vi "TLB Native Dynamic Events ver 0.26.vi"() -> ()   [LabVIEW 2018] (continued)
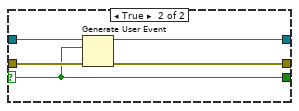
[diagram p2: hidden frame]
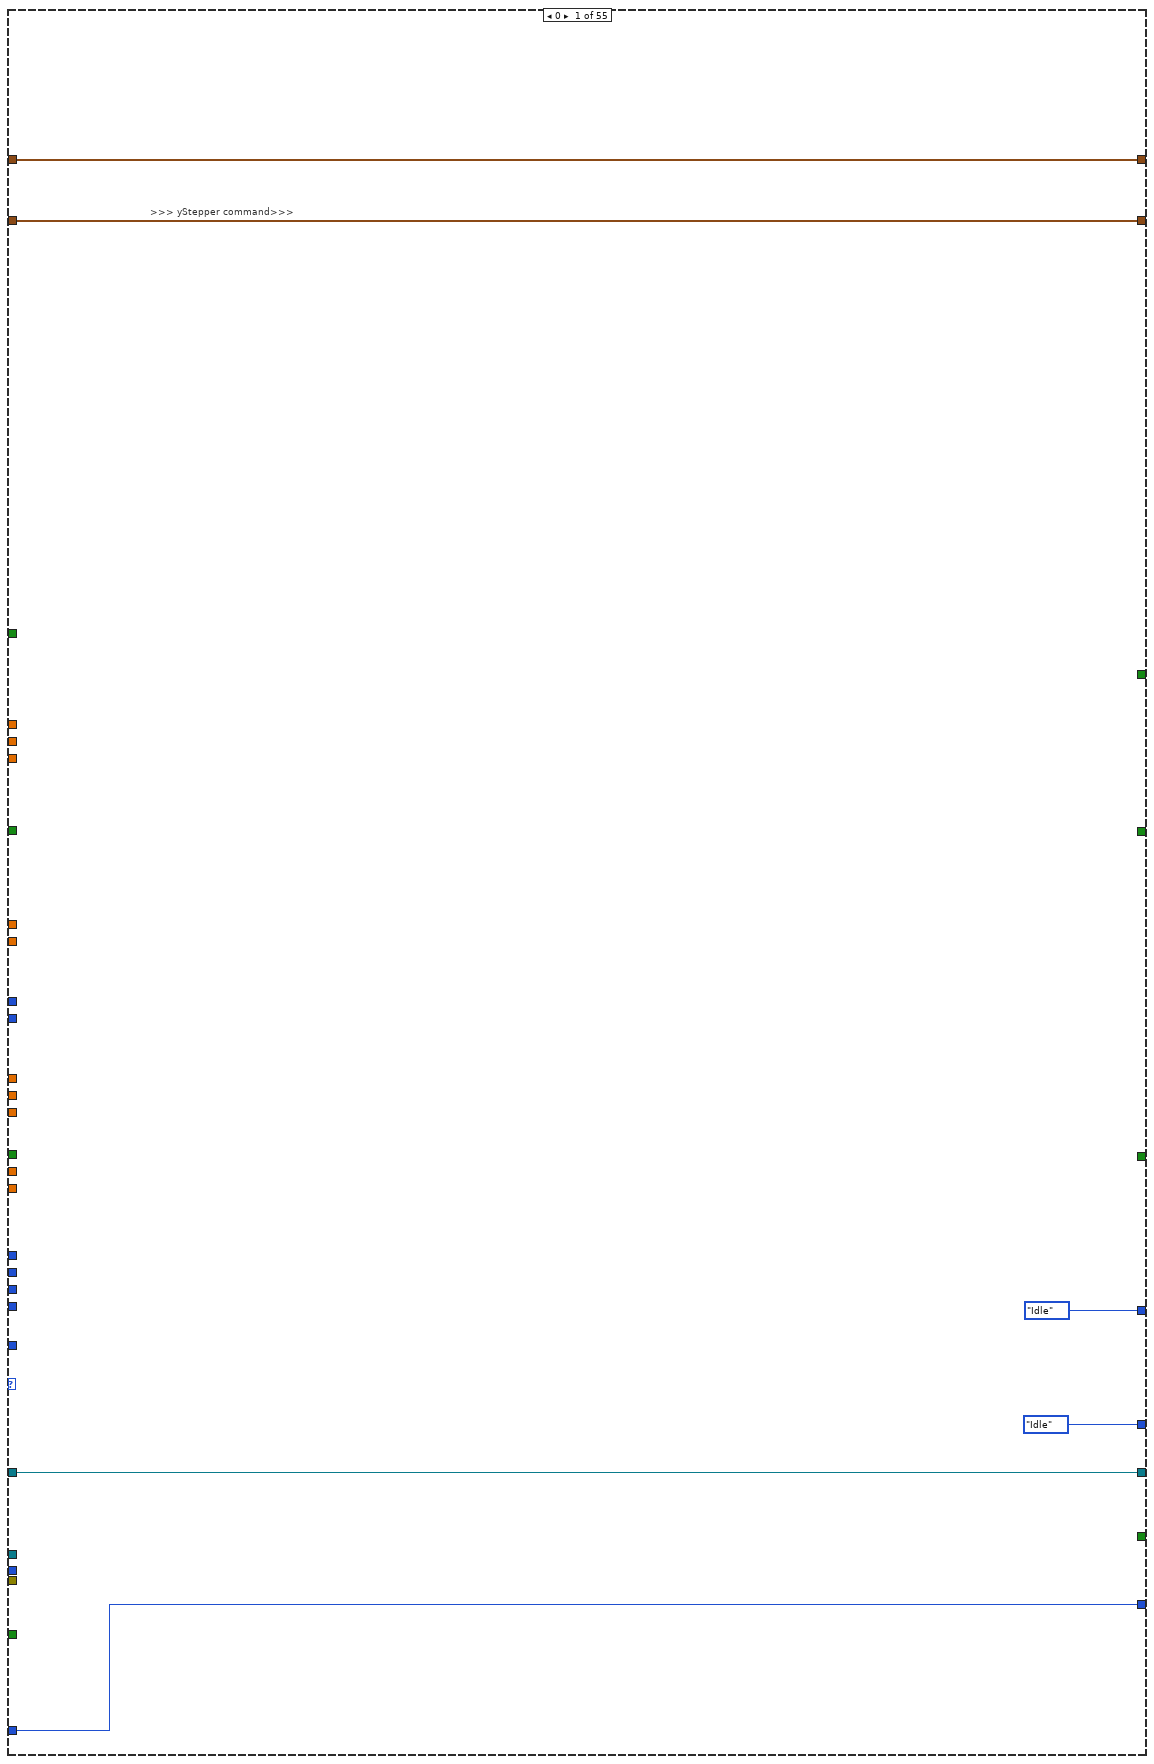
[diagram p5: hidden frame]
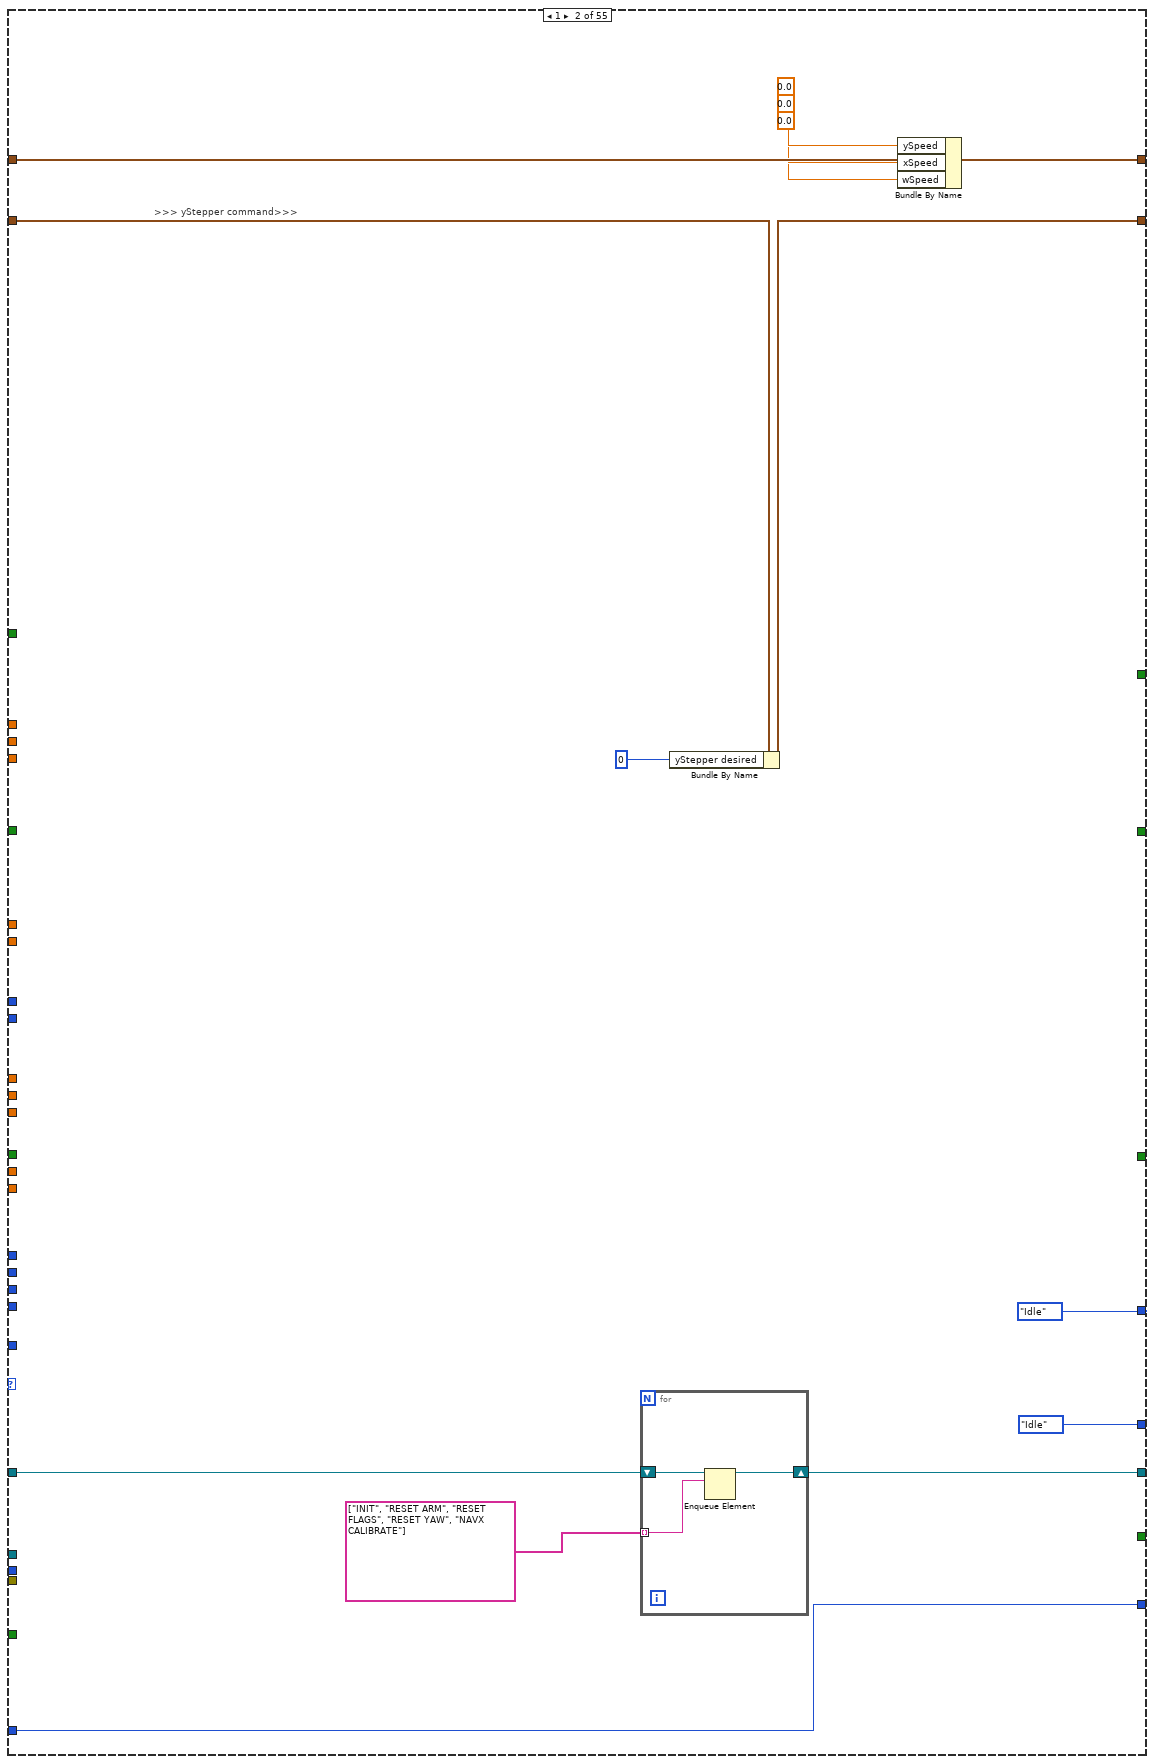
[diagram p6: hidden frame]
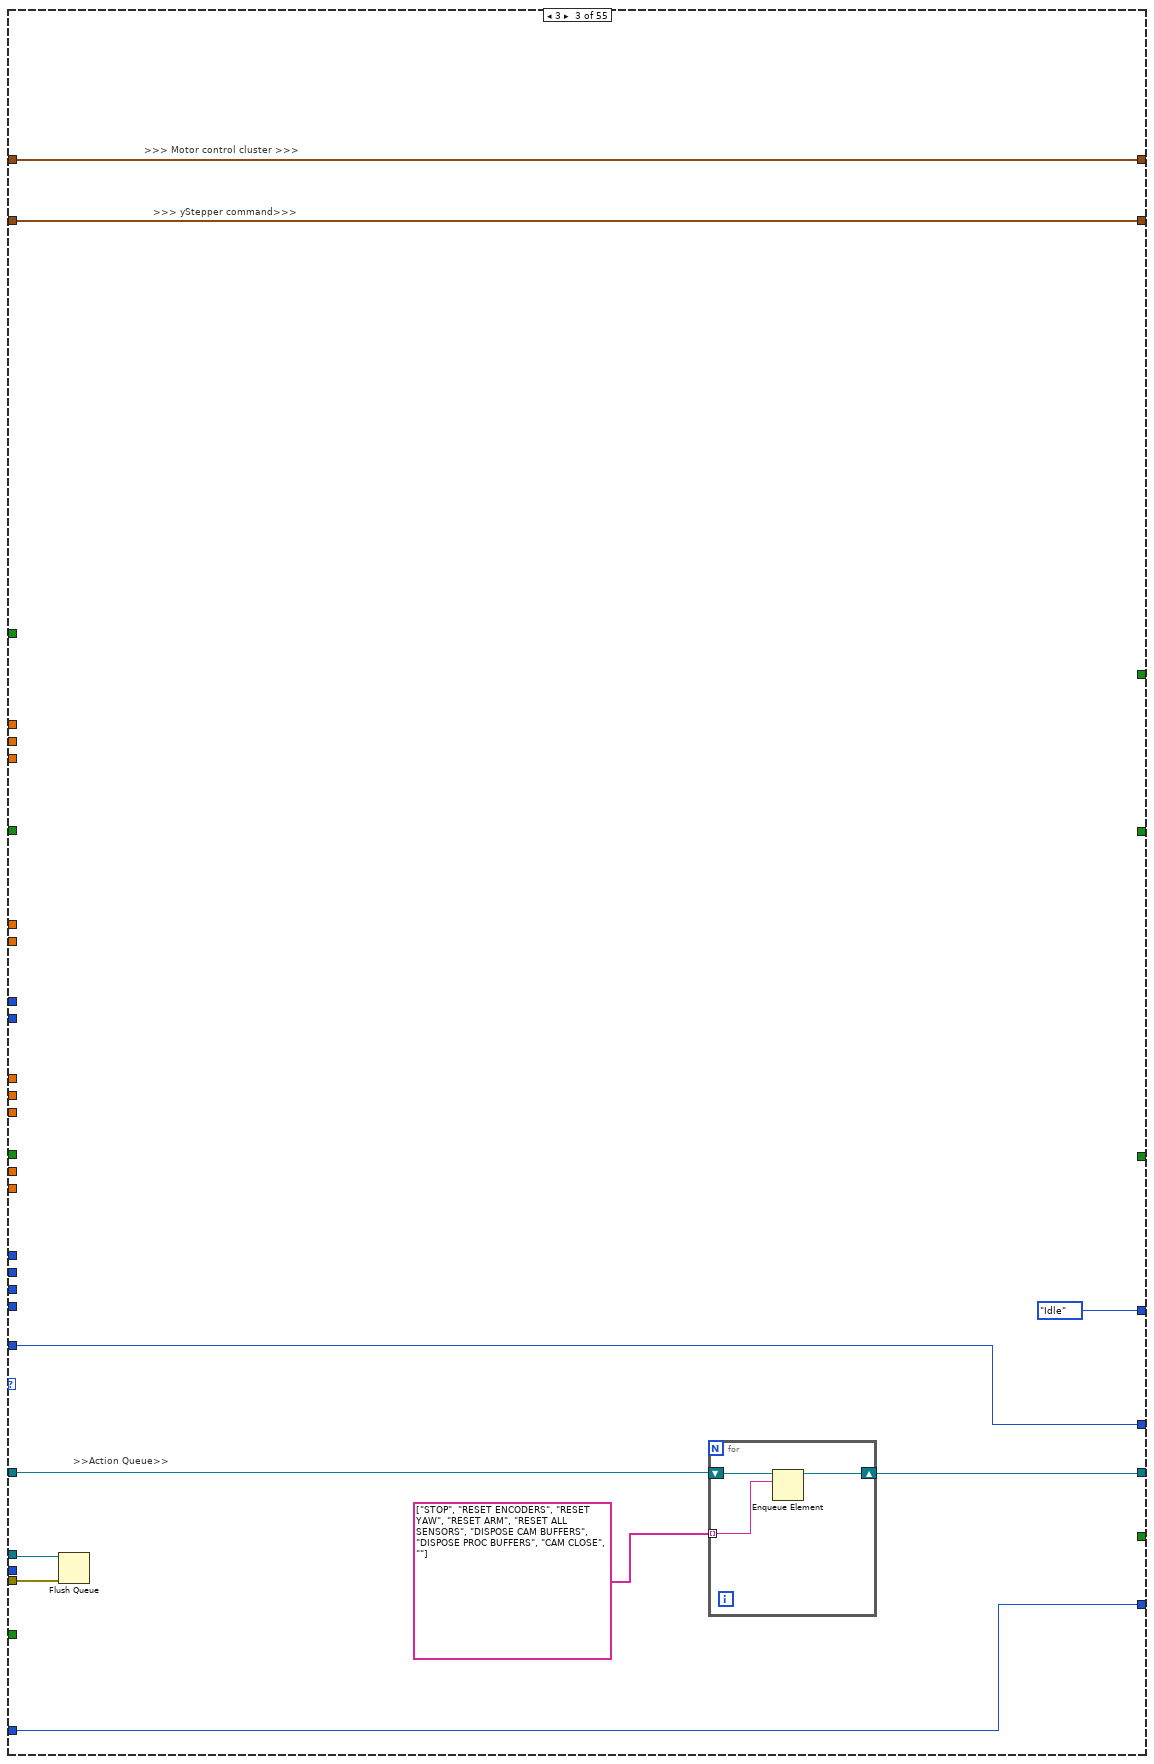
[diagram p7: hidden frame]
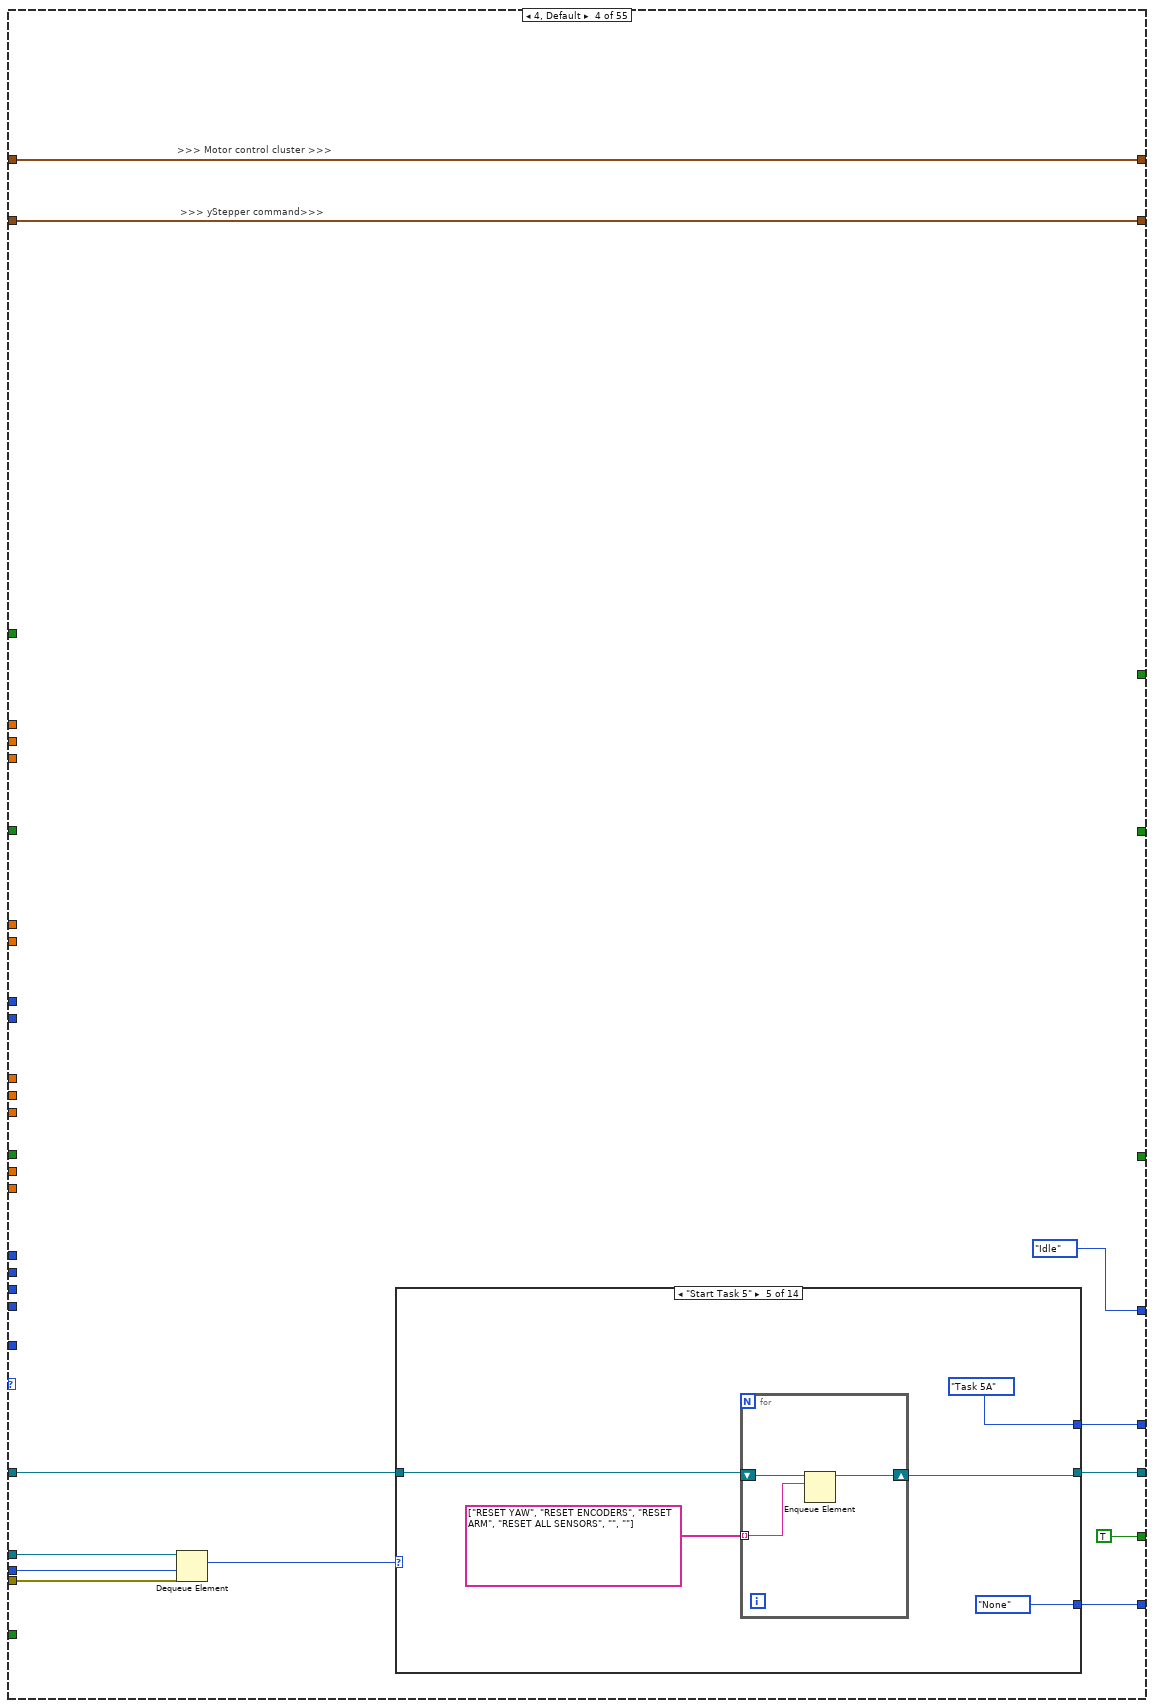
[diagram p8: hidden frame]
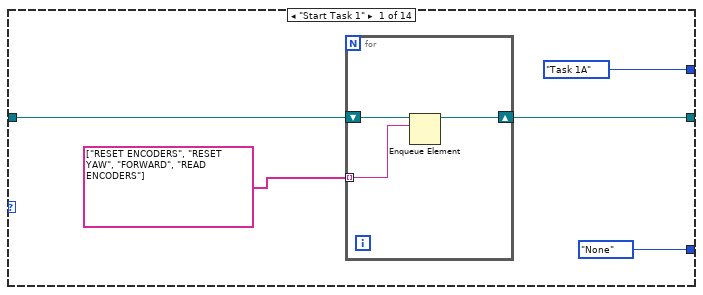
[diagram p9: hidden frame]
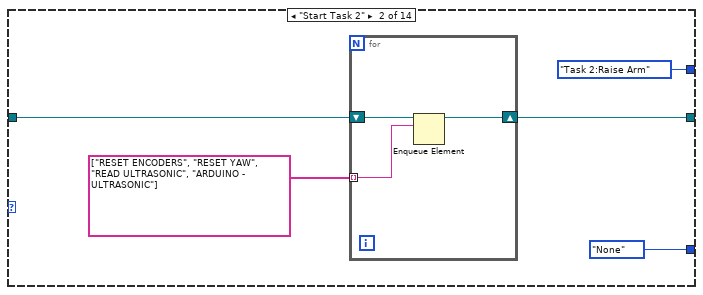
[diagram p10: hidden frame]
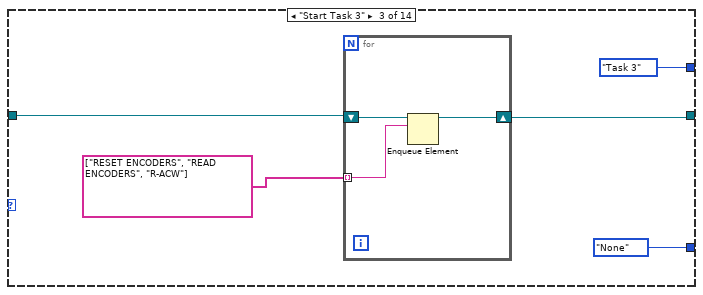
[diagram p11: hidden frame]
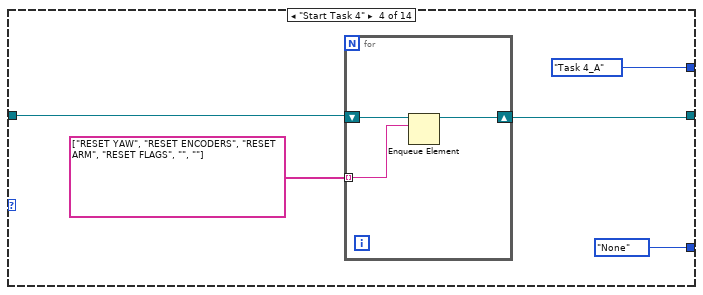
[diagram p12: hidden frame]
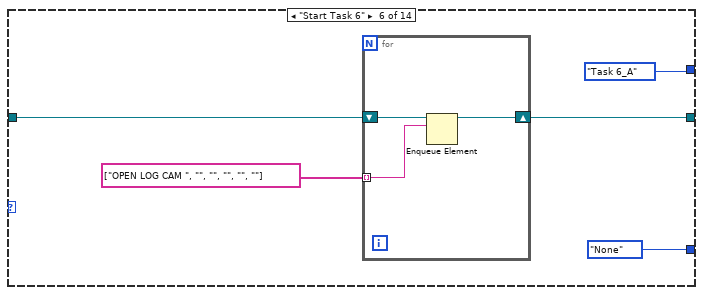
[diagram p13: hidden frame]
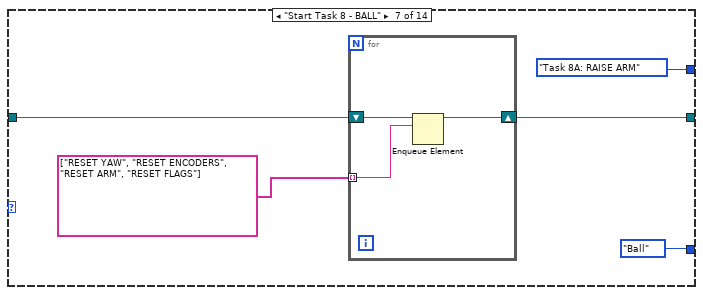
[diagram p14: hidden frame]
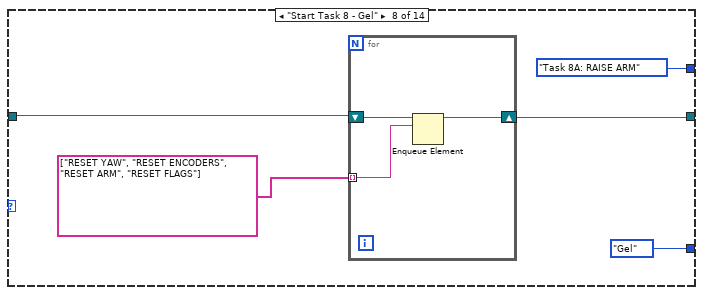
[diagram p15: hidden frame]
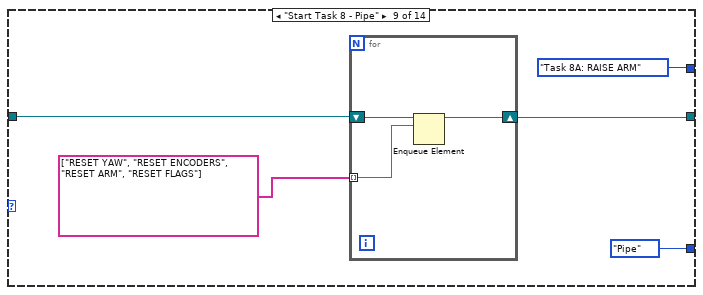
[diagram p16: hidden frame]
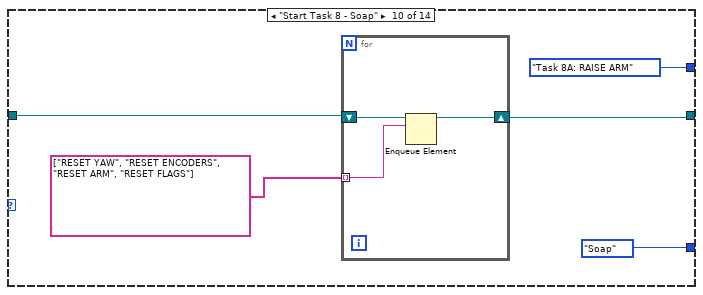
[diagram p17: hidden frame]
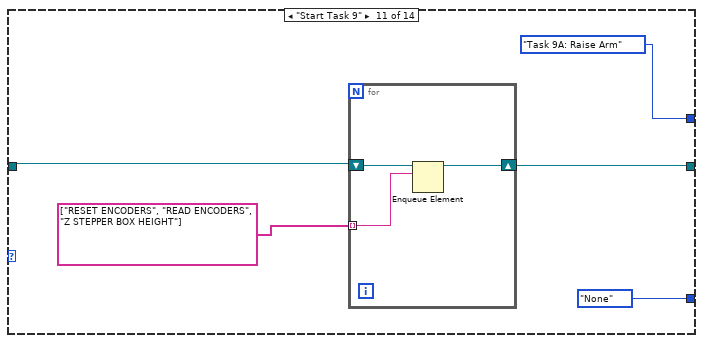
[diagram p18: hidden frame]
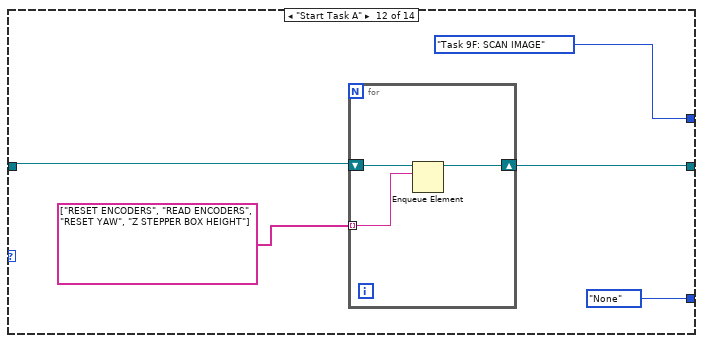
[diagram p19: hidden frame]
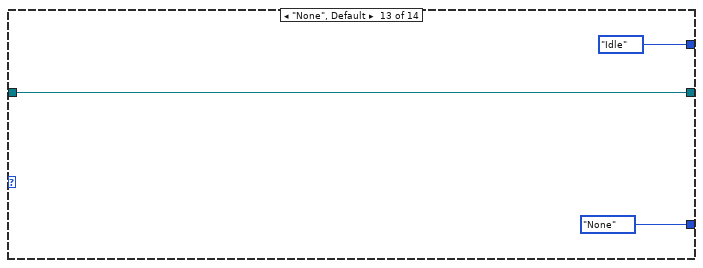
[diagram p20: hidden frame]
                      shift-left: w2521 -> [w2524]
                      n813 = Enqueue Element(queue=w2524, element=w2523) -> (queue out=w2525:refnum<queue>)  [unwired: 2 in, 2 out]
                    }
                  }
                  frame True {
                    n814 = for {
                      shift-right: [w2530] -> w2527
                      shift-left: w2528 -> [w2531]
                      tunnel: string[] ["STOP", "RESET ENCODERS", "RESET YAW", "OPEN LIFE CAM", "SET TIMER 2", "RESET FLAGS"] -> [w2529] mode=indexing
                      n815 = Enqueue Element(queue=w2531, element=w2529) -> (queue out=w2530:refnum<queue>)  [unwired: 2 in, 2 out]
                    }
                  }
                }
                n816 = Or(x=w2511, y=w2510) -> (x .or. y?=w2509:bool)
                n817 = Select(t=State_Type_Definitions,_for_0.26g_versions_and_later_2."True Stop" ("Enum"), s=w2510, f=State_Type_Definitions."Task 9N: SCAN IMAGE" ("Enum")) -> (s? t:f=w2512:u16)
                n818 = Select(t=w2512, s=w2509, f=State_Type_Definitions,_for_0.26g_versions_and_later_2."Task 9M: MOVE RIGHT" ("Enum")) -> (s? t:f=w2518:u16)
              }
              frame "Exit" {
                n819 = for {
                  shift-right: [w2538] -> w2535
                  shift-left: w2534 -> [w2539]
                  tunnel: string[] ["STOP", "RESET ENCODERS", "RESET YAW", "ARDUINO MODE 0"] -> [w2537] mode=indexing
                  n820 = Enqueue Element(queue=w2539, element=w2537) -> (queue out=w2538:refnum<queue>)  [unwired: 2 in, 2 out]
                }
              }
            }
          }
          frame 51 {
            # ">> Manual override >>"
            n821 = Dequeue Element(queue=w2548, timeout in ms (-1)=w2547, error in (no error)=w2546) -> (element=w2549:T8)  [unwired: 3 out]
            n822 = case shown="\"Start Task 1\", Default" w2549 {
              tunnel: [w2563 State_Type_Definitions,_for_0.26g_versions_and_later_2."True Stop" ("Enum")] -> w2541
              tunnel: [w2561 w2579] -> w2540
              tunnel: w2544 -> [w2560 w2576]
              tunnel: w2545 -> [w2554 _]
              tunnel: [State_Type_Definitions,_for_0.26g_versions_and_later_2."Idle" ("Enum") State_Type_Definitions,_for_0.26g_versions_and_later_2."Shutdown" ("Enum")] -> w2542
              tunnel: w2543 -> [w2553 _]
              frame "Start Task 1", Default {
                # ">> WIill proceed to part ii if not manual override >>"
                # ">>If ENABLE or Trigger is set to true>>"
                n823 = Or(x=w2553, y=w2554) -> (x .or. y?=w2555:bool)
                n824 = case shown="False" w2553 {
                  tunnel: [w2566 w2572] -> w2561
                  tunnel: w2560 -> [w2565 w2571]
                  frame False {
                    n825 = for {
                      shift-right: [w2568] -> w2566
                      shift-left: w2565 -> [w2569]
                      tunnel: string[] ["CAM ACQ", "START TIMER"] ("element") -> [w2567] mode=indexing
                      n826 = Enqueue Element(queue=w2569, element=w2567) -> (queue out=w2568:refnum<queue>)  [unwired: 2 in, 2 out]
                    }
                  }
                  frame True {
                    n827 = for {
                      shift-right: [w2574] -> w2572
                      shift-left: w2571 -> [w2575]
                      tunnel: string[] ["CLOSE CAM", "SET TIMER 5", "", "", "", ""] -> [w2573] mode=indexing
                      n828 = Enqueue Element(queue=w2575, element=w2573) -> (queue out=w2574:refnum<queue>)  [unwired: 2 in, 2 out]
                    }
                  }
                }
                n829 = Select(t=State_Type_Definitions,_for_0.26g_versions_and_later_2."True Stop" ("Enum"), s=w2554, f=State_Type_Definitions."Task 9O: PROCESS COLOUR" ("Enum")) -> (s? t:f=w2557:u16)
                n830 = Select(t=w2557, s=w2555, f=State_Type_Definitions."Task 9N: SCAN IMAGE" ("Enum")) -> (s? t:f=w2563:u16)
              }
              frame "Exit" {
                n831 = for {
                  shift-right: [w2582] -> w2579
                  shift-left: w2576 -> [w2583]
                  tunnel: string[] ["STOP", "RESET ENCODERS", "RESET YAW", ""] -> [w2581] mode=indexing
                  n832 = Enqueue Element(queue=w2583, element=w2581) -> (queue out=w2582:refnum<queue>)  [unwired: 2 in, 2 out]
                }
              }
            }
          }
          frame 52 {
            # ">> Item Selection Bias >>"
            n833 = Dequeue Element(queue=w2591, timeout in ms (-1)=w2590, error in (no error)=w2589) -> (element=w2593:T8)  [unwired: 3 out]
            n834 = case shown="\"Start Task 1\", Default" w2593 {
              tunnel: w2584 -> [w2599 _]
              tunnel: [w2606 State_Type_Definitions,_for_0.26g_versions_and_later_2."True Stop" ("Enum")] -> w2587
              tunnel: w2588 -> [w2598 _]
              tunnel: w2592 -> [w2605 w2622]
              tunnel: [w2604 w2623] -> w2586
              tunnel: [State_Type_Definitions,_for_0.26g_versions_and_later_2."Idle" ("Enum") State_Type_Definitions,_for_0.26g_versions_and_later_2."Shutdown" ("Enum")] -> w2585
              frame "Start Task 1", Default {
                n835 = case shown="False" w2599 {
                  tunnel: w2605 -> [w2609 w2616]
                  tunnel: [w2610 w2615] -> w2604
                  frame False {
                    n836 = for {
                      tunnel: string[] ["START TIMER", "COLOUR PROCESSING", ""] ("element") -> [w2611] mode=indexing
                      shift-right: [w2613] -> w2610
                      shift-left: w2609 -> [w2612]
                      n837 = Enqueue Element(queue=w2612, element=w2611) -> (queue out=w2613:refnum<queue>)  [unwired: 2 in, 2 out]
                    }
                  }
                  frame True {
                    n838 = for {
                      shift-right: [w2618] -> w2615
                      shift-left: w2616 -> [w2619]
                      tunnel: string[] ["CLOSE CAM", "DISPOSE BUFFERS", "RESET ENCODERS", "RESET YAW", "RESET FLAGS", ""] -> [w2617] mode=indexing
                      n839 = Enqueue Element(queue=w2619, element=w2617) -> (queue out=w2618:refnum<queue>)  [unwired: 2 in, 2 out]
                    }
                  }
                }
                n840 = Or(x=w2599, y=w2598) -> (x .or. y?=w2597:bool)
                n841 = Select(t=State_Type_Definitions,_for_0.26g_versions_and_later_2."True Stop" ("Enum"), s=w2598, f=State_Type_Definitions."Task 9P: MOVE RIGHT" ("Enum")) -> (s? t:f=w2600:u16)
                n842 = Select(t=w2600, s=w2597, f=State_Type_Definitions."Task 9O: PROCESS COLOUR" ("Enum")) -> (s? t:f=w2606:u16)
              }
              frame "Exit" {
                n843 = for {
                  shift-right: [w2626] -> w2623
                  shift-left: w2622 -> [w2627]
                  tunnel: string[] ["STOP", "RESET ENCODERS", "RESET YAW", "ARDUINO MODE 0"] -> [w2625] mode=indexing
                  n844 = Enqueue Element(queue=w2627, element=w2625) -> (queue out=w2626:refnum<queue>)  [unwired: 2 in, 2 out]
                }
              }
            }
          }
          frame 53 {
            # ">> Item Selection Bias >>"
            n845 = Dequeue Element(queue=w2633, timeout in ms (-1)=w2632, error in (no error)=w2631) -> (element=w2641:T8)  [unwired: 3 out]
            n846 = Greater?(x=w2629, y=50.0) -> (0:w2639:bool)
            n847 = And(x=w2628, y=w2639) -> (x .and. y?=w2640:bool)
            n848 = case shown="\"Start Task 1\", Default" w2641 {
              tunnel: w2640 -> [w2647 _]
              tunnel: [w2654 State_Type_Definitions,_for_0.26g_versions_and_later_2."True Stop" ("Enum")] -> w2636
              tunnel: w2630 -> [w2646 _]
              tunnel: w2634 -> [w2653 w2670]
              tunnel: [w2652 w2671] -> w2635
              tunnel: [State_Type_Definitions,_for_0.26g_versions_and_later_2."Idle" ("Enum") State_Type_Definitions,_for_0.26g_versions_and_later_2."Shutdown" ("Enum")] -> w2637
              frame "Start Task 1", Default {
                n849 = case shown="False" w2647 {
                  tunnel: w2653 -> [w2657 w2664]
                  tunnel: [w2658 w2663] -> w2652
                  frame False {
                    n850 = for {
                      tunnel: string[] ["READ LINE SENSOR", "READ NAVX", "RIGHT", "READ ENCODERS"] ("element") -> [w2659] mode=indexing
                      shift-right: [w2661] -> w2658
                      shift-left: w2657 -> [w2660]
                      n851 = Enqueue Element(queue=w2660, element=w2659) -> (queue out=w2661:refnum<queue>)  [unwired: 2 in, 2 out]
                    }
                  }
                  frame True {
                    n852 = for {
                      shift-right: [w2666] -> w2663
                      shift-left: w2664 -> [w2667]
                      tunnel: string[] ["STOP", "RESET ENCODERS", "RESET YAW", "OPEN LIFE CAM", "SET TIMER 2", "RESET FLAGS"] -> [w2665] mode=indexing
                      n853 = Enqueue Element(queue=w2667, element=w2665) -> (queue out=w2666:refnum<queue>)  [unwired: 2 in, 2 out]
                    }
                  }
                }
                n854 = Or(x=w2647, y=w2646) -> (x .or. y?=w2645:bool)
                n855 = Select(t=State_Type_Definitions,_for_0.26g_versions_and_later_2."True Stop" ("Enum"), s=w2646, f=State_Type_Definitions."Task 9Q: SCAN IMAGE" ("Enum")) -> (s? t:f=w2648:u16)
                n856 = Select(t=w2648, s=w2645, f=State_Type_Definitions."Task 9P: MOVE RIGHT" ("Enum")) -> (s? t:f=w2654:u16)
              }
              frame "Exit" {
                n857 = for {
                  shift-right: [w2674] -> w2671
                  shift-left: w2670 -> [w2675]
                  tunnel: string[] ["STOP", "RESET ENCODERS", "RESET YAW", "ARDUINO MODE 0"] -> [w2673] mode=indexing
                  n858 = Enqueue Element(queue=w2675, element=w2673) -> (queue out=w2674:refnum<queue>)  [unwired: 2 in, 2 out]
                }
              }
            }
          }
          frame 54 {
            # ">> Manual override >>"
            n859 = Dequeue Element(queue=w2684, timeout in ms (-1)=w2683, error in (no error)=w2682) -> (element=w2685:T8)  [unwired: 3 out]
            n860 = case shown="\"Start Task 1\", Default" w2685 {
              tunnel: [w2699 State_Type_Definitions,_for_0.26g_versions_and_later_2."True Stop" ("Enum")] -> w2677
              tunnel: [w2697 w2715] -> w2676
              tunnel: w2680 -> [w2696 w2712]
              tunnel: w2681 -> [w2690 _]
              tunnel: [State_Type_Definitions,_for_0.26g_versions_and_later_2."Idle" ("Enum") State_Type_Definitions,_for_0.26g_versions_and_later_2."Shutdown" ("Enum")] -> w2678
              tunnel: w2679 -> [w2689 _]
              frame "Start Task 1", Default {
                # ">> WIill proceed to part ii if not manual override >>"
                # ">>If ENABLE or Trigger is set to true>>"
                n861 = Or(x=w2689, y=w2690) -> (x .or. y?=w2691:bool)
                n862 = case shown="False" w2689 {
                  tunnel: [w2702 w2708] -> w2697
                  tunnel: w2696 -> [w2701 w2707]
                  frame False {
                    n863 = for {
                      shift-right: [w2704] -> w2702
                      shift-left: w2701 -> [w2705]
                      tunnel: string[] ["CAM ACQ", "START TIMER"] ("element") -> [w2703] mode=indexing
                      n864 = Enqueue Element(queue=w2705, element=w2703) -> (queue out=w2704:refnum<queue>)  [unwired: 2 in, 2 out]
                    }
                  }
                  frame True {
                    n865 = for {
                      shift-right: [w2710] -> w2708
                      shift-left: w2707 -> [w2711]
                      tunnel: string[] ["CLOSE CAM", "SET TIMER 5", "", "", "", ""] -> [w2709] mode=indexing
                      n866 = Enqueue Element(queue=w2711, element=w2709) -> (queue out=w2710:refnum<queue>)  [unwired: 2 in, 2 out]
                    }
                  }
                }
                n867 = Select(t=State_Type_Definitions,_for_0.26g_versions_and_later_2."True Stop" ("Enum"), s=w2690, f=State_Type_Definitions,_for_0.26g_versions_and_later_2."Task 9R: PROCESS COLOUR" ("Enum")) -> (s? t:f=w2693:T16)
                n868 = Select(t=w2693, s=w2691, f=State_Type_Definitions."Task 9Q: SCAN IMAGE" ("Enum")) -> (s? t:f=w2699:u16)
              }
              frame "Exit" {
                n869 = for {
                  shift-right: [w2718] -> w2715
                  shift-left: w2712 -> [w2719]
                  tunnel: string[] ["STOP", "RESET ENCODERS", "RESET YAW", ""] -> [w2717] mode=indexing
                  n870 = Enqueue Element(queue=w2719, element=w2717) -> (queue out=w2718:refnum<queue>)  [unwired: 2 in, 2 out]
                }
              }
            }
          }
          frame 55 {
            # ">> Item Selection Bias >>"
            # ">>> Motor control cluster >>>"
            # ">>> yStepper command>>>"
            n871 = Dequeue Element(queue=w2725, timeout in ms (-1)=w2726, error in (no error)=w2727) -> (element=w2729:T8)  [unwired: 3 out]
            n872 = case shown="\"Start Task 1\", Default" w2729 {
              tunnel: w2723 -> [w2735 _]
              tunnel: [w2742 State_Type_Definitions,_for_0.26g_versions_and_later_2."True Stop" ("Enum")] -> w2721
              tunnel: w2728 -> [w2734 _]
              tunnel: w2724 -> [w2741 w2758]
              tunnel: [w2740 w2759] -> w2720
              tunnel: [State_Type_Definitions,_for_0.26g_versions_and_later_2."Idle" ("Enum") State_Type_Definitions,_for_0.26g_versions_and_later_2."Shutdown" ("Enum")] -> w2722
              frame "Start Task 1", Default {
                n873 = case shown="False" w2735 {
                  tunnel: w2741 -> [w2745 w2752]
                  tunnel: [w2746 w2751] -> w2740
                  frame False {
                    n874 = for {
                      tunnel: string[] ["START TIMER", "COLOUR PROCESSING", ""] ("element") -> [w2747] mode=indexing
                      shift-right: [w2749] -> w2746
                      shift-left: w2745 -> [w2748]
                      n875 = Enqueue Element(queue=w2748, element=w2747) -> (queue out=w2749:refnum<queue>)  [unwired: 2 in, 2 out]
                    }
                  }
                  frame True {
                    n876 = for {
                      shift-right: [w2754] -> w2751
                      shift-left: w2752 -> [w2755]
                      tunnel: string[] ["CLOSE CAM", "DISPOSE BUFFERS", "RESET ENCODERS", "RESET YAW", "RESET FLAGS", ""] -> [w2753] mode=indexing
                      n877 = Enqueue Element(queue=w2755, element=w2753) -> (queue out=w2754:refnum<queue>)  [unwired: 2 in, 2 out]
                    }
                  }
                }
                n878 = Or(x=w2735, y=w2734) -> (x .or. y?=w2733:bool)
                n879 = Select(t=State_Type_Definitions,_for_0.26g_versions_and_later_2."True Stop" ("Enum"), s=w2734, f=State_Type_Definitions,_for_0.26g_versions_and_later_2."True Stop" ("Enum")) -> (s? t:f=w2736:T16)
                n880 = Select(t=w2736, s=w2733, f=State_Type_Definitions,_for_0.26g_versions_and_later_2."Task 9R: PROCESS COLOUR" ("Enum")) -> (s? t:f=w2742:T16)
              }
              frame "Exit" {
                n881 = for {
                  shift-right: [w2762] -> w2759
                  shift-left: w2758 -> [w2763]
                  tunnel: string[] ["STOP", "RESET ENCODERS", "RESET YAW", "ARDUINO MODE 0"] -> [w2761] mode=indexing
                  n882 = Enqueue Element(queue=w2763, element=w2761) -> (queue out=w2762:refnum<queue>)  [unwired: 2 in, 2 out]
                }
              }
            }
          }
        }
        "Object Detection" <- w307
        "Ultrasonic sensors" <- w330
        "Encoder values" <- w319
        "Stepper position values" <- w303
        "NAVX Values" <- w301
        "IR Sensors" <- w293
        "Line sensors" <- w288
        "Time cluster" <- w299
      }
    }
    "Object recognition mode" <- w215
    "Front Ultrasonic obstruct" <- w212
    "Front IR obstruct" <- w211
    "Table IR obstruct" <- w210
    n883 = local write "Green LED"(w225) -> ()
  }
  n884 = while {
    stop <- w3528 stop-if-true
    n885 = call "MOTOR CONTROL WITH PID AE.vi"("AE Mode"=MOTOR_CONTROL_WITH_PID_AE_DATA_MODE_TYPE_DEF."Read from AE") -> ("Speed & distance"=→"Speed & distance":T13)  [unwired: 3 in]
    n886 = call "FGV Stop.vi"("Init/Read/Write State"=States_for_Action_Engine."Read") -> ("Output node"=w3528:bool)  [unwired: 2 in, 1 out]
    n887 = Wait (ms)(milliseconds to wait=u32 5) -> ()  [unwired: 1 out]
  }
  n888 = call <vilib>:"DIO Close.vi"("error in (no error)"=w22, "DIO Info In"=w25) -> ()  [unwired: 9 in, 1 out]
  n889 = call <vilib>:"DIO Close.vi"("error in (no error)"=w32, "DIO Info In"=w34) -> ()  [unwired: 9 in, 1 out]
  n890 = call <vilib>:"NavX Close.vi"("error in (no error)"=w9, "NavX Info In"=w8) -> ()  [unwired: 9 in, 1 out]
  n891 = call <vilib>:"DIO Close.vi"("error in (no error)"=w27, "DIO Info In"=w29) -> ()  [unwired: 9 in, 1 out]
  n892 = call <vilib>:"DIO Close.vi"("error in (no error)"=w16, "DIO Info In"=w17) -> ()  [unwired: 9 in, 1 out]
  n893 = call <vilib>:"DIO Close.vi"("error in (no error)"=w11, "DIO Info In"=w12) -> ()  [unwired: 9 in, 1 out]
  n894 = Merge Errors "Merge Errors"(w62, w61) -> (w44:errorcluster)
  n895 = Merge Errors(w48, w44) -> (w43:errorcluster)
  n896 = Destroy User Event(user event=w66, error in=w43) -> ()  [unwired: 1 out]
  n897 = Release Queue(queue=w39, error in (no error)=w43) -> (error out=→"Queue Errors":errorcluster)  [unwired: 1 in, 2 out]
  n898 = Release Queue(queue=w56, error in (no error)=w43) -> ()  [unwired: 1 in, 3 out]
  n899 = Destroy User Event(user event=w65, error in=w43) -> ()  [unwired: 1 out]
  n900 = Unregister For Events(event registration refnum=w57, error in=w43) -> ()  [unwired: 1 out]
